vi "run_pharmaBotExp_v0.015.vi"(0 "data in":T12={"daq_ao 1"="Dev1/ao0", "daq_ai 1"="Dev1/ai0", "experiment day folder"=path "C:/multiBot/data/debug/testing", "Multiclamp init error"=0, "Multiclamp Handle Out"=10225184, "sampling rate (Hz)"=20000, "trial name"="t1"}, 1 "auto run?":bool=TRUE, 3 "which manipulator":T13(ring), 4 "HEK/slice options":enum16{"slice", "HEK"}(ring), 5 "error in":errorcluster, 6 "Validate after Experiment":bool, 7 "common cluster":T9, 11 "individual controls in":T8, 13 "images":T3={"slice image"="remote image 000000001461186C", "pipette template"="remote image 000000001461152C", "found pipette"=refnum, "pipette mask for cell tracker"=refnum, "cell images ref"=refnum}) -> (10 "Cell Looks Good?":bool=TRUE, 12 "ValidationOutputCluster":T5(array[cluster]), 14 "ValidationResults":waveform(dbl)[][](array[waveform]), 15 "ValidationPos1":T6(array[ring]), 16 "Exp. Terminated":bool, 17 "ValidationPos2":T6(array[ring]), 18 "ValidationWaveform":waveform(dbl)[](array[waveform]), 19 "error out":errorcluster)   [LabVIEW 2015] (continued)
              tunnel: w1798 -> [_ _ _ _ _ _ _ _ _ w1834 _ _ _ _ _]
              tunnel: w1797 -> [_ _ _ _ _ _ _ _ _ _ w1837 _ _ _ _]
              tunnel: w1796 -> [_ _ _ _ _ _ _ _ _ _ _ w1840 _ _ _]
              tunnel: w1795 -> [_ _ _ _ _ _ _ _ _ _ _ _ w1843 _ _]
              frame "False", Default {
              }
              frame "Single Jump" {
                n1386 = property class="TabCtl (strict)"(reference=w1811, "Value"=w1810) -> ()  [unwired: 1 in, 2 out]
                n1387 = property class="TabCtl (strict)"(reference=w1811, "Visible"=TRUE) -> ()  [unwired: 1 in, 2 out]
              }
              frame "Solution Change" {
                n1388 = property class="TabCtl (strict)"(reference=w1814, "Visible"=TRUE) -> ()  [unwired: 1 in, 2 out]
                n1389 = property class="TabCtl (strict)"(reference=w1814, "Value"=w1813) -> ()  [unwired: 1 in, 2 out]
              }
              frame "Voltage Step" {
                n1390 = property class="TabCtl (strict)"(reference=w1817, "Value"=w1816) -> ()  [unwired: 1 in, 2 out]
                n1391 = property class="TabCtl (strict)"(reference=w1817, "Visible"=TRUE) -> ()  [unwired: 1 in, 2 out]
              }
              frame "Voltage Ramp" {
                n1392 = property class="TabCtl (strict)"(reference=w1820, "Value"=w1819) -> ()  [unwired: 1 in, 2 out]
                n1393 = property class="TabCtl (strict)"(reference=w1820, "Visible"=TRUE) -> ()  [unwired: 1 in, 2 out]
              }
              frame "Voltage Pulse" {
                n1394 = property class="TabCtl (strict)"(reference=w1823, "Value"=w1822) -> ()  [unwired: 1 in, 2 out]
                n1395 = property class="TabCtl (strict)"(reference=w1823, "Visible"=TRUE) -> ()  [unwired: 1 in, 2 out]
              }
              frame "Jump Train" {
                n1396 = property class="TabCtl (strict)"(reference=w1826, "Value"=w1825) -> ()  [unwired: 1 in, 2 out]
                n1397 = property class="TabCtl (strict)"(reference=w1826, "Visible"=TRUE) -> ()  [unwired: 1 in, 2 out]
              }
              frame "Paired Pulse" {
                n1398 = property class="TabCtl (strict)"(reference=w1829, "Value"=w1828) -> ()  [unwired: 1 in, 2 out]
                n1399 = property class="TabCtl (strict)"(reference=w1829, "Visible"=TRUE) -> ()  [unwired: 1 in, 2 out]
              }
              frame "Single Manip Jump" {
                n1400 = property class="TabCtl (strict)"(reference=w1832, "Value"=w1831) -> ()  [unwired: 1 in, 2 out]
                n1401 = property class="TabCtl (strict)"(reference=w1832, "Visible"=TRUE) -> ()  [unwired: 1 in, 2 out]
              }
              frame "Gap Free" {
                n1402 = property class="TabCtl (strict)"(reference=w1835, "Value"=w1834) -> ()  [unwired: 1 in, 2 out]
                n1403 = property class="TabCtl (strict)"(reference=w1835, "Visible"=TRUE) -> ()  [unwired: 1 in, 2 out]
              }
              frame "Gap Free Iclamp" {
                n1404 = property class="TabCtl (strict)"(reference=w1838, "Value"=w1837) -> ()  [unwired: 1 in, 2 out]
                n1405 = property class="TabCtl (strict)"(reference=w1838, "Visible"=TRUE) -> ()  [unwired: 1 in, 2 out]
              }
              frame "Current Pulse" {
                n1406 = property class="TabCtl (strict)"(reference=w1841, "Value"=w1840) -> ()  [unwired: 1 in, 2 out]
                n1407 = property class="TabCtl (strict)"(reference=w1841, "Visible"=TRUE) -> ()  [unwired: 1 in, 2 out]
              }
              frame "Current Ramp" {
                n1408 = property class="TabCtl (strict)"(reference=w1844, "Value"=w1843) -> ()  [unwired: 1 in, 2 out]
                n1409 = property class="TabCtl (strict)"(reference=w1844, "Visible"=TRUE) -> ()  [unwired: 1 in, 2 out]
              }
              frame "Multi M. Jump" {
                n1410 = property class="TabCtl (strict)"(reference=w1847, "Value"=w1846) -> ()  [unwired: 1 in, 2 out]
                n1411 = property class="TabCtl (strict)"(reference=w1847, "Visible"=TRUE) -> ()  [unwired: 1 in, 2 out]
              }
              frame "none" {
                n1412 = property class="TabCtl (strict)"(reference=w1849, "Visible"=FALSE) -> ()  [unwired: 1 in, 2 out]
              }
            }
          }
          frame "PhaseC Experiment Option" {
            n1413 = control-ref of="Experiment Selection C"() -> (w1864:refnum<vi>)
            n1414 = case shown="\"Current Ramp\"" w1865 {
              tunnel: w1864 -> [_ w1867 w1870 w1873 w1876 w1879 w1882 w1885 w1888 w1891 w1894 w1897 w1900 w1903 w1905]
              tunnel: w1863 -> [_ _ _ _ _ _ _ _ _ _ _ _ _ w1902 _]
              tunnel: w1862 -> [_ w1866 _ _ _ _ _ _ _ _ _ _ _ _ _]
              tunnel: w1861 -> [_ _ w1869 _ _ _ _ _ _ _ _ _ _ _ _]
              tunnel: w1860 -> [_ _ _ w1872 _ _ _ _ _ _ _ _ _ _ _]
              tunnel: w1859 -> [_ _ _ _ w1875 _ _ _ _ _ _ _ _ _ _]
              tunnel: w1858 -> [_ _ _ _ _ w1878 _ _ _ _ _ _ _ _ _]
              tunnel: w1857 -> [_ _ _ _ _ _ w1881 _ _ _ _ _ _ _ _]
              tunnel: w1856 -> [_ _ _ _ _ _ _ w1884 _ _ _ _ _ _ _]
              tunnel: w1855 -> [_ _ _ _ _ _ _ _ w1887 _ _ _ _ _ _]
              tunnel: w1854 -> [_ _ _ _ _ _ _ _ _ w1890 _ _ _ _ _]
              tunnel: w1853 -> [_ _ _ _ _ _ _ _ _ _ w1893 _ _ _ _]
              tunnel: w1852 -> [_ _ _ _ _ _ _ _ _ _ _ w1896 _ _ _]
              tunnel: w1851 -> [_ _ _ _ _ _ _ _ _ _ _ _ w1899 _ _]
              frame "False", Default {
              }
              frame "Single Jump" {
                n1415 = property class="TabCtl (strict)"(reference=w1867, "Value"=w1866) -> ()  [unwired: 1 in, 2 out]
                n1416 = property class="TabCtl (strict)"(reference=w1867, "Visible"=TRUE) -> ()  [unwired: 1 in, 2 out]
              }
              frame "Solution Change" {
                n1417 = property class="TabCtl (strict)"(reference=w1870, "Visible"=TRUE) -> ()  [unwired: 1 in, 2 out]
                n1418 = property class="TabCtl (strict)"(reference=w1870, "Value"=w1869) -> ()  [unwired: 1 in, 2 out]
              }
              frame "Voltage Step" {
                n1419 = property class="TabCtl (strict)"(reference=w1873, "Value"=w1872) -> ()  [unwired: 1 in, 2 out]
                n1420 = property class="TabCtl (strict)"(reference=w1873, "Visible"=TRUE) -> ()  [unwired: 1 in, 2 out]
              }
              frame "Voltage Ramp" {
                n1421 = property class="TabCtl (strict)"(reference=w1876, "Value"=w1875) -> ()  [unwired: 1 in, 2 out]
                n1422 = property class="TabCtl (strict)"(reference=w1876, "Visible"=TRUE) -> ()  [unwired: 1 in, 2 out]
              }
              frame "Voltage Pulse" {
                n1423 = property class="TabCtl (strict)"(reference=w1879, "Value"=w1878) -> ()  [unwired: 1 in, 2 out]
                n1424 = property class="TabCtl (strict)"(reference=w1879, "Visible"=TRUE) -> ()  [unwired: 1 in, 2 out]
              }
              frame "Jump Train" {
                n1425 = property class="TabCtl (strict)"(reference=w1882, "Value"=w1881) -> ()  [unwired: 1 in, 2 out]
                n1426 = property class="TabCtl (strict)"(reference=w1882, "Visible"=TRUE) -> ()  [unwired: 1 in, 2 out]
              }
              frame "Paired Pulse" {
                n1427 = property class="TabCtl (strict)"(reference=w1885, "Value"=w1884) -> ()  [unwired: 1 in, 2 out]
                n1428 = property class="TabCtl (strict)"(reference=w1885, "Visible"=TRUE) -> ()  [unwired: 1 in, 2 out]
              }
              frame "Single Manip Jump" {
                n1429 = property class="TabCtl (strict)"(reference=w1888, "Value"=w1887) -> ()  [unwired: 1 in, 2 out]
                n1430 = property class="TabCtl (strict)"(reference=w1888, "Visible"=TRUE) -> ()  [unwired: 1 in, 2 out]
              }
              frame "Gap Free" {
                n1431 = property class="TabCtl (strict)"(reference=w1891, "Value"=w1890) -> ()  [unwired: 1 in, 2 out]
                n1432 = property class="TabCtl (strict)"(reference=w1891, "Visible"=TRUE) -> ()  [unwired: 1 in, 2 out]
              }
              frame "Gap Free Iclamp" {
                n1433 = property class="TabCtl (strict)"(reference=w1894, "Value"=w1893) -> ()  [unwired: 1 in, 2 out]
                n1434 = property class="TabCtl (strict)"(reference=w1894, "Visible"=TRUE) -> ()  [unwired: 1 in, 2 out]
              }
              frame "Current Pulse" {
                n1435 = property class="TabCtl (strict)"(reference=w1897, "Value"=w1896) -> ()  [unwired: 1 in, 2 out]
                n1436 = property class="TabCtl (strict)"(reference=w1897, "Visible"=TRUE) -> ()  [unwired: 1 in, 2 out]
              }
              frame "Current Ramp" {
                n1437 = property class="TabCtl (strict)"(reference=w1900, "Value"=w1899) -> ()  [unwired: 1 in, 2 out]
                n1438 = property class="TabCtl (strict)"(reference=w1900, "Visible"=TRUE) -> ()  [unwired: 1 in, 2 out]
              }
              frame "Multi M. Jump" {
                n1439 = property class="TabCtl (strict)"(reference=w1903, "Value"=w1902) -> ()  [unwired: 1 in, 2 out]
                n1440 = property class="TabCtl (strict)"(reference=w1903, "Visible"=TRUE) -> ()  [unwired: 1 in, 2 out]
              }
              frame "none" {
                n1441 = property class="TabCtl (strict)"(reference=w1905, "Visible"=FALSE) -> ()  [unwired: 1 in, 2 out]
              }
            }
          }
          frame "PhaseD Experiment Option" {
            n1442 = control-ref of="Experiment Selection D"() -> (w1920:refnum<vi>)
            n1443 = case shown="\"Current Ramp\"" w1921 {
              tunnel: w1920 -> [_ w1923 w1926 w1929 w1932 w1935 w1938 w1941 w1944 w1947 w1950 w1953 w1956 w1959 w1961]
              tunnel: w1919 -> [_ _ _ _ _ _ _ _ _ _ _ _ _ w1958 _]
              tunnel: w1918 -> [_ w1922 _ _ _ _ _ _ _ _ _ _ _ _ _]
              tunnel: w1917 -> [_ _ w1925 _ _ _ _ _ _ _ _ _ _ _ _]
              tunnel: w1916 -> [_ _ _ w1928 _ _ _ _ _ _ _ _ _ _ _]
              tunnel: w1915 -> [_ _ _ _ w1931 _ _ _ _ _ _ _ _ _ _]
              tunnel: w1914 -> [_ _ _ _ _ w1934 _ _ _ _ _ _ _ _ _]
              tunnel: w1913 -> [_ _ _ _ _ _ w1937 _ _ _ _ _ _ _ _]
              tunnel: w1912 -> [_ _ _ _ _ _ _ w1940 _ _ _ _ _ _ _]
              tunnel: w1911 -> [_ _ _ _ _ _ _ _ w1943 _ _ _ _ _ _]
              tunnel: w1910 -> [_ _ _ _ _ _ _ _ _ w1946 _ _ _ _ _]
              tunnel: w1909 -> [_ _ _ _ _ _ _ _ _ _ w1949 _ _ _ _]
              tunnel: w1908 -> [_ _ _ _ _ _ _ _ _ _ _ w1952 _ _ _]
              tunnel: w1907 -> [_ _ _ _ _ _ _ _ _ _ _ _ w1955 _ _]
              frame "False", Default {
              }
              frame "Single Jump" {
                n1444 = property class="TabCtl (strict)"(reference=w1923, "Value"=w1922) -> ()  [unwired: 1 in, 2 out]
                n1445 = property class="TabCtl (strict)"(reference=w1923, "Visible"=TRUE) -> ()  [unwired: 1 in, 2 out]
              }
              frame "Solution Change" {
                n1446 = property class="TabCtl (strict)"(reference=w1926, "Visible"=TRUE) -> ()  [unwired: 1 in, 2 out]
                n1447 = property class="TabCtl (strict)"(reference=w1926, "Value"=w1925) -> ()  [unwired: 1 in, 2 out]
              }
              frame "Voltage Step" {
                n1448 = property class="TabCtl (strict)"(reference=w1929, "Value"=w1928) -> ()  [unwired: 1 in, 2 out]
                n1449 = property class="TabCtl (strict)"(reference=w1929, "Visible"=TRUE) -> ()  [unwired: 1 in, 2 out]
              }
              frame "Voltage Ramp" {
                n1450 = property class="TabCtl (strict)"(reference=w1932, "Value"=w1931) -> ()  [unwired: 1 in, 2 out]
                n1451 = property class="TabCtl (strict)"(reference=w1932, "Visible"=TRUE) -> ()  [unwired: 1 in, 2 out]
              }
              frame "Voltage Pulse" {
                n1452 = property class="TabCtl (strict)"(reference=w1935, "Value"=w1934) -> ()  [unwired: 1 in, 2 out]
                n1453 = property class="TabCtl (strict)"(reference=w1935, "Visible"=TRUE) -> ()  [unwired: 1 in, 2 out]
              }
              frame "Jump Train" {
                n1454 = property class="TabCtl (strict)"(reference=w1938, "Value"=w1937) -> ()  [unwired: 1 in, 2 out]
                n1455 = property class="TabCtl (strict)"(reference=w1938, "Visible"=TRUE) -> ()  [unwired: 1 in, 2 out]
              }
              frame "Paired Pulse" {
                n1456 = property class="TabCtl (strict)"(reference=w1941, "Value"=w1940) -> ()  [unwired: 1 in, 2 out]
                n1457 = property class="TabCtl (strict)"(reference=w1941, "Visible"=TRUE) -> ()  [unwired: 1 in, 2 out]
              }
              frame "Single Manip Jump" {
                n1458 = property class="TabCtl (strict)"(reference=w1944, "Value"=w1943) -> ()  [unwired: 1 in, 2 out]
                n1459 = property class="TabCtl (strict)"(reference=w1944, "Visible"=TRUE) -> ()  [unwired: 1 in, 2 out]
              }
              frame "Gap Free" {
                n1460 = property class="TabCtl (strict)"(reference=w1947, "Value"=w1946) -> ()  [unwired: 1 in, 2 out]
                n1461 = property class="TabCtl (strict)"(reference=w1947, "Visible"=TRUE) -> ()  [unwired: 1 in, 2 out]
              }
              frame "Gap Free Iclamp" {
                n1462 = property class="TabCtl (strict)"(reference=w1950, "Value"=w1949) -> ()  [unwired: 1 in, 2 out]
                n1463 = property class="TabCtl (strict)"(reference=w1950, "Visible"=TRUE) -> ()  [unwired: 1 in, 2 out]
              }
              frame "Current Pulse" {
                n1464 = property class="TabCtl (strict)"(reference=w1953, "Value"=w1952) -> ()  [unwired: 1 in, 2 out]
                n1465 = property class="TabCtl (strict)"(reference=w1953, "Visible"=TRUE) -> ()  [unwired: 1 in, 2 out]
              }
              frame "Current Ramp" {
                n1466 = property class="TabCtl (strict)"(reference=w1956, "Value"=w1955) -> ()  [unwired: 1 in, 2 out]
                n1467 = property class="TabCtl (strict)"(reference=w1956, "Visible"=TRUE) -> ()  [unwired: 1 in, 2 out]
              }
              frame "Multi M. Jump" {
                n1468 = property class="TabCtl (strict)"(reference=w1959, "Value"=w1958) -> ()  [unwired: 1 in, 2 out]
                n1469 = property class="TabCtl (strict)"(reference=w1959, "Visible"=TRUE) -> ()  [unwired: 1 in, 2 out]
              }
              frame "none" {
                n1470 = property class="TabCtl (strict)"(reference=w1961, "Visible"=FALSE) -> ()  [unwired: 1 in, 2 out]
              }
            }
          }
          frame "PhaseE Experiment Option" {
            n1471 = control-ref of="Experiment Selection E"() -> (w1976:refnum<vi>)
            n1472 = case shown="\"Current Ramp\"" w1977 {
              tunnel: w1976 -> [_ w1979 w1982 w1985 w1988 w1991 w1994 w1997 w2000 w2003 w2006 w2009 w2012 w2015 w2017]
              tunnel: w1975 -> [_ _ _ _ _ _ _ _ _ _ _ _ _ w2014 _]
              tunnel: w1974 -> [_ w1978 _ _ _ _ _ _ _ _ _ _ _ _ _]
              tunnel: w1973 -> [_ _ w1981 _ _ _ _ _ _ _ _ _ _ _ _]
              tunnel: w1972 -> [_ _ _ w1984 _ _ _ _ _ _ _ _ _ _ _]
              tunnel: w1971 -> [_ _ _ _ w1987 _ _ _ _ _ _ _ _ _ _]
              tunnel: w1970 -> [_ _ _ _ _ w1990 _ _ _ _ _ _ _ _ _]
              tunnel: w1969 -> [_ _ _ _ _ _ w1993 _ _ _ _ _ _ _ _]
              tunnel: w1968 -> [_ _ _ _ _ _ _ w1996 _ _ _ _ _ _ _]
              tunnel: w1967 -> [_ _ _ _ _ _ _ _ w1999 _ _ _ _ _ _]
              tunnel: w1966 -> [_ _ _ _ _ _ _ _ _ w2002 _ _ _ _ _]
              tunnel: w1965 -> [_ _ _ _ _ _ _ _ _ _ w2005 _ _ _ _]
              tunnel: w1964 -> [_ _ _ _ _ _ _ _ _ _ _ w2008 _ _ _]
              tunnel: w1963 -> [_ _ _ _ _ _ _ _ _ _ _ _ w2011 _ _]
              frame "False", Default {
              }
              frame "Single Jump" {
                n1473 = property class="TabCtl (strict)"(reference=w1979, "Value"=w1978) -> ()  [unwired: 1 in, 2 out]
                n1474 = property class="TabCtl (strict)"(reference=w1979, "Visible"=TRUE) -> ()  [unwired: 1 in, 2 out]
              }
              frame "Solution Change" {
                n1475 = property class="TabCtl (strict)"(reference=w1982, "Visible"=TRUE) -> ()  [unwired: 1 in, 2 out]
                n1476 = property class="TabCtl (strict)"(reference=w1982, "Value"=w1981) -> ()  [unwired: 1 in, 2 out]
              }
              frame "Voltage Step" {
                n1477 = property class="TabCtl (strict)"(reference=w1985, "Value"=w1984) -> ()  [unwired: 1 in, 2 out]
                n1478 = property class="TabCtl (strict)"(reference=w1985, "Visible"=TRUE) -> ()  [unwired: 1 in, 2 out]
              }
              frame "Voltage Ramp" {
                n1479 = property class="TabCtl (strict)"(reference=w1988, "Value"=w1987) -> ()  [unwired: 1 in, 2 out]
                n1480 = property class="TabCtl (strict)"(reference=w1988, "Visible"=TRUE) -> ()  [unwired: 1 in, 2 out]
              }
              frame "Voltage Pulse" {
                n1481 = property class="TabCtl (strict)"(reference=w1991, "Value"=w1990) -> ()  [unwired: 1 in, 2 out]
                n1482 = property class="TabCtl (strict)"(reference=w1991, "Visible"=TRUE) -> ()  [unwired: 1 in, 2 out]
              }
              frame "Jump Train" {
                n1483 = property class="TabCtl (strict)"(reference=w1994, "Value"=w1993) -> ()  [unwired: 1 in, 2 out]
                n1484 = property class="TabCtl (strict)"(reference=w1994, "Visible"=TRUE) -> ()  [unwired: 1 in, 2 out]
              }
              frame "Paired Pulse" {
                n1485 = property class="TabCtl (strict)"(reference=w1997, "Value"=w1996) -> ()  [unwired: 1 in, 2 out]
                n1486 = property class="TabCtl (strict)"(reference=w1997, "Visible"=TRUE) -> ()  [unwired: 1 in, 2 out]
              }
              frame "Single Manip Jump" {
                n1487 = property class="TabCtl (strict)"(reference=w2000, "Value"=w1999) -> ()  [unwired: 1 in, 2 out]
                n1488 = property class="TabCtl (strict)"(reference=w2000, "Visible"=TRUE) -> ()  [unwired: 1 in, 2 out]
              }
              frame "Gap Free" {
                n1489 = property class="TabCtl (strict)"(reference=w2003, "Value"=w2002) -> ()  [unwired: 1 in, 2 out]
                n1490 = property class="TabCtl (strict)"(reference=w2003, "Visible"=TRUE) -> ()  [unwired: 1 in, 2 out]
              }
              frame "Gap Free Iclamp" {
                n1491 = property class="TabCtl (strict)"(reference=w2006, "Value"=w2005) -> ()  [unwired: 1 in, 2 out]
                n1492 = property class="TabCtl (strict)"(reference=w2006, "Visible"=TRUE) -> ()  [unwired: 1 in, 2 out]
              }
              frame "Current Pulse" {
                n1493 = property class="TabCtl (strict)"(reference=w2009, "Value"=w2008) -> ()  [unwired: 1 in, 2 out]
                n1494 = property class="TabCtl (strict)"(reference=w2009, "Visible"=TRUE) -> ()  [unwired: 1 in, 2 out]
              }
              frame "Current Ramp" {
                n1495 = property class="TabCtl (strict)"(reference=w2012, "Value"=w2011) -> ()  [unwired: 1 in, 2 out]
                n1496 = property class="TabCtl (strict)"(reference=w2012, "Visible"=TRUE) -> ()  [unwired: 1 in, 2 out]
              }
              frame "Multi M. Jump" {
                n1497 = property class="TabCtl (strict)"(reference=w2015, "Value"=w2014) -> ()  [unwired: 1 in, 2 out]
                n1498 = property class="TabCtl (strict)"(reference=w2015, "Visible"=TRUE) -> ()  [unwired: 1 in, 2 out]
              }
              frame "none" {
                n1499 = property class="TabCtl (strict)"(reference=w2017, "Visible"=FALSE) -> ()  [unwired: 1 in, 2 out]
              }
            }
          }
          frame "PhaseF Experiment Option" {
            n1500 = control-ref of="Experiment Selection F"() -> (w2032:refnum<vi>)
            n1501 = case shown="\"Current Ramp\"" w2033 {
              tunnel: w2032 -> [_ w2035 w2038 w2041 w2044 w2047 w2050 w2053 w2056 w2059 w2062 w2065 w2068 w2071 w2073]
              tunnel: w2031 -> [_ _ _ _ _ _ _ _ _ _ _ _ _ w2070 _]
              tunnel: w2030 -> [_ w2034 _ _ _ _ _ _ _ _ _ _ _ _ _]
              tunnel: w2029 -> [_ _ w2037 _ _ _ _ _ _ _ _ _ _ _ _]
              tunnel: w2028 -> [_ _ _ w2040 _ _ _ _ _ _ _ _ _ _ _]
              tunnel: w2027 -> [_ _ _ _ w2043 _ _ _ _ _ _ _ _ _ _]
              tunnel: w2026 -> [_ _ _ _ _ w2046 _ _ _ _ _ _ _ _ _]
              tunnel: w2025 -> [_ _ _ _ _ _ w2049 _ _ _ _ _ _ _ _]
              tunnel: w2024 -> [_ _ _ _ _ _ _ w2052 _ _ _ _ _ _ _]
              tunnel: w2023 -> [_ _ _ _ _ _ _ _ w2055 _ _ _ _ _ _]
              tunnel: w2022 -> [_ _ _ _ _ _ _ _ _ w2058 _ _ _ _ _]
              tunnel: w2021 -> [_ _ _ _ _ _ _ _ _ _ w2061 _ _ _ _]
              tunnel: w2020 -> [_ _ _ _ _ _ _ _ _ _ _ w2064 _ _ _]
              tunnel: w2019 -> [_ _ _ _ _ _ _ _ _ _ _ _ w2067 _ _]
              frame "False", Default {
              }
              frame "Single Jump" {
                n1502 = property class="TabCtl (strict)"(reference=w2035, "Value"=w2034) -> ()  [unwired: 1 in, 2 out]
                n1503 = property class="TabCtl (strict)"(reference=w2035, "Visible"=TRUE) -> ()  [unwired: 1 in, 2 out]
              }
              frame "Solution Change" {
                n1504 = property class="TabCtl (strict)"(reference=w2038, "Visible"=TRUE) -> ()  [unwired: 1 in, 2 out]
                n1505 = property class="TabCtl (strict)"(reference=w2038, "Value"=w2037) -> ()  [unwired: 1 in, 2 out]
              }
              frame "Voltage Step" {
                n1506 = property class="TabCtl (strict)"(reference=w2041, "Value"=w2040) -> ()  [unwired: 1 in, 2 out]
                n1507 = property class="TabCtl (strict)"(reference=w2041, "Visible"=TRUE) -> ()  [unwired: 1 in, 2 out]
              }
              frame "Voltage Ramp" {
                n1508 = property class="TabCtl (strict)"(reference=w2044, "Value"=w2043) -> ()  [unwired: 1 in, 2 out]
                n1509 = property class="TabCtl (strict)"(reference=w2044, "Visible"=TRUE) -> ()  [unwired: 1 in, 2 out]
              }
              frame "Voltage Pulse" {
                n1510 = property class="TabCtl (strict)"(reference=w2047, "Value"=w2046) -> ()  [unwired: 1 in, 2 out]
                n1511 = property class="TabCtl (strict)"(reference=w2047, "Visible"=TRUE) -> ()  [unwired: 1 in, 2 out]
              }
              frame "Jump Train" {
                n1512 = property class="TabCtl (strict)"(reference=w2050, "Value"=w2049) -> ()  [unwired: 1 in, 2 out]
                n1513 = property class="TabCtl (strict)"(reference=w2050, "Visible"=TRUE) -> ()  [unwired: 1 in, 2 out]
              }
              frame "Paired Pulse" {
                n1514 = property class="TabCtl (strict)"(reference=w2053, "Value"=w2052) -> ()  [unwired: 1 in, 2 out]
                n1515 = property class="TabCtl (strict)"(reference=w2053, "Visible"=TRUE) -> ()  [unwired: 1 in, 2 out]
              }
              frame "Single Manip Jump" {
                n1516 = property class="TabCtl (strict)"(reference=w2056, "Value"=w2055) -> ()  [unwired: 1 in, 2 out]
                n1517 = property class="TabCtl (strict)"(reference=w2056, "Visible"=TRUE) -> ()  [unwired: 1 in, 2 out]
              }
              frame "Gap Free" {
                n1518 = property class="TabCtl (strict)"(reference=w2059, "Value"=w2058) -> ()  [unwired: 1 in, 2 out]
                n1519 = property class="TabCtl (strict)"(reference=w2059, "Visible"=TRUE) -> ()  [unwired: 1 in, 2 out]
              }
              frame "Gap Free Iclamp" {
                n1520 = property class="TabCtl (strict)"(reference=w2062, "Value"=w2061) -> ()  [unwired: 1 in, 2 out]
                n1521 = property class="TabCtl (strict)"(reference=w2062, "Visible"=TRUE) -> ()  [unwired: 1 in, 2 out]
              }
              frame "Current Pulse" {
                n1522 = property class="TabCtl (strict)"(reference=w2065, "Value"=w2064) -> ()  [unwired: 1 in, 2 out]
                n1523 = property class="TabCtl (strict)"(reference=w2065, "Visible"=TRUE) -> ()  [unwired: 1 in, 2 out]
              }
              frame "Current Ramp" {
                n1524 = property class="TabCtl (strict)"(reference=w2068, "Value"=w2067) -> ()  [unwired: 1 in, 2 out]
                n1525 = property class="TabCtl (strict)"(reference=w2068, "Visible"=TRUE) -> ()  [unwired: 1 in, 2 out]
              }
              frame "Multi M. Jump" {
                n1526 = property class="TabCtl (strict)"(reference=w2071, "Value"=w2070) -> ()  [unwired: 1 in, 2 out]
                n1527 = property class="TabCtl (strict)"(reference=w2071, "Visible"=TRUE) -> ()  [unwired: 1 in, 2 out]
              }
              frame "none" {
                n1528 = property class="TabCtl (strict)"(reference=w2073, "Visible"=FALSE) -> ()  [unwired: 1 in, 2 out]
              }
            }
          }
          frame "PhaseG Experiment Option" {
            n1529 = control-ref of="Experiment Selection G"() -> (w2088:refnum<vi>)
            n1530 = case shown="\"Current Ramp\"" w2089 {
              tunnel: w2088 -> [_ w2091 w2094 w2097 w2100 w2103 w2106 w2109 w2112 w2115 w2118 w2121 w2124 w2127 w2129]
              tunnel: w2087 -> [_ _ _ _ _ _ _ _ _ _ _ _ _ w2126 _]
              tunnel: w2086 -> [_ w2090 _ _ _ _ _ _ _ _ _ _ _ _ _]
              tunnel: w2085 -> [_ _ w2093 _ _ _ _ _ _ _ _ _ _ _ _]
              tunnel: w2084 -> [_ _ _ w2096 _ _ _ _ _ _ _ _ _ _ _]
              tunnel: w2083 -> [_ _ _ _ w2099 _ _ _ _ _ _ _ _ _ _]
              tunnel: w2082 -> [_ _ _ _ _ w2102 _ _ _ _ _ _ _ _ _]
              tunnel: w2081 -> [_ _ _ _ _ _ w2105 _ _ _ _ _ _ _ _]
              tunnel: w2080 -> [_ _ _ _ _ _ _ w2108 _ _ _ _ _ _ _]
              tunnel: w2079 -> [_ _ _ _ _ _ _ _ w2111 _ _ _ _ _ _]
              tunnel: w2078 -> [_ _ _ _ _ _ _ _ _ w2114 _ _ _ _ _]
              tunnel: w2077 -> [_ _ _ _ _ _ _ _ _ _ w2117 _ _ _ _]
              tunnel: w2076 -> [_ _ _ _ _ _ _ _ _ _ _ w2120 _ _ _]
              tunnel: w2075 -> [_ _ _ _ _ _ _ _ _ _ _ _ w2123 _ _]
              frame "False", Default {
              }
              frame "Single Jump" {
                n1531 = property class="TabCtl (strict)"(reference=w2091, "Value"=w2090) -> ()  [unwired: 1 in, 2 out]
                n1532 = property class="TabCtl (strict)"(reference=w2091, "Visible"=TRUE) -> ()  [unwired: 1 in, 2 out]
              }
              frame "Solution Change" {
                n1533 = property class="TabCtl (strict)"(reference=w2094, "Visible"=TRUE) -> ()  [unwired: 1 in, 2 out]
                n1534 = property class="TabCtl (strict)"(reference=w2094, "Value"=w2093) -> ()  [unwired: 1 in, 2 out]
              }
              frame "Voltage Step" {
                n1535 = property class="TabCtl (strict)"(reference=w2097, "Value"=w2096) -> ()  [unwired: 1 in, 2 out]
                n1536 = property class="TabCtl (strict)"(reference=w2097, "Visible"=TRUE) -> ()  [unwired: 1 in, 2 out]
              }
              frame "Voltage Ramp" {
                n1537 = property class="TabCtl (strict)"(reference=w2100, "Value"=w2099) -> ()  [unwired: 1 in, 2 out]
                n1538 = property class="TabCtl (strict)"(reference=w2100, "Visible"=TRUE) -> ()  [unwired: 1 in, 2 out]
              }
              frame "Voltage Pulse" {
                n1539 = property class="TabCtl (strict)"(reference=w2103, "Value"=w2102) -> ()  [unwired: 1 in, 2 out]
                n1540 = property class="TabCtl (strict)"(reference=w2103, "Visible"=TRUE) -> ()  [unwired: 1 in, 2 out]
              }
              frame "Jump Train" {
                n1541 = property class="TabCtl (strict)"(reference=w2106, "Value"=w2105) -> ()  [unwired: 1 in, 2 out]
                n1542 = property class="TabCtl (strict)"(reference=w2106, "Visible"=TRUE) -> ()  [unwired: 1 in, 2 out]
              }
              frame "Paired Pulse" {
                n1543 = property class="TabCtl (strict)"(reference=w2109, "Value"=w2108) -> ()  [unwired: 1 in, 2 out]
                n1544 = property class="TabCtl (strict)"(reference=w2109, "Visible"=TRUE) -> ()  [unwired: 1 in, 2 out]
              }
              frame "Single Manip Jump" {
                n1545 = property class="TabCtl (strict)"(reference=w2112, "Value"=w2111) -> ()  [unwired: 1 in, 2 out]
                n1546 = property class="TabCtl (strict)"(reference=w2112, "Visible"=TRUE) -> ()  [unwired: 1 in, 2 out]
              }
              frame "Gap Free" {
                n1547 = property class="TabCtl (strict)"(reference=w2115, "Value"=w2114) -> ()  [unwired: 1 in, 2 out]
                n1548 = property class="TabCtl (strict)"(reference=w2115, "Visible"=TRUE) -> ()  [unwired: 1 in, 2 out]
              }
              frame "Gap Free Iclamp" {
                n1549 = property class="TabCtl (strict)"(reference=w2118, "Value"=w2117) -> ()  [unwired: 1 in, 2 out]
                n1550 = property class="TabCtl (strict)"(reference=w2118, "Visible"=TRUE) -> ()  [unwired: 1 in, 2 out]
              }
              frame "Current Pulse" {
                n1551 = property class="TabCtl (strict)"(reference=w2121, "Value"=w2120) -> ()  [unwired: 1 in, 2 out]
                n1552 = property class="TabCtl (strict)"(reference=w2121, "Visible"=TRUE) -> ()  [unwired: 1 in, 2 out]
              }
              frame "Current Ramp" {
                n1553 = property class="TabCtl (strict)"(reference=w2124, "Value"=w2123) -> ()  [unwired: 1 in, 2 out]
                n1554 = property class="TabCtl (strict)"(reference=w2124, "Visible"=TRUE) -> ()  [unwired: 1 in, 2 out]
              }
              frame "Multi M. Jump" {
                n1555 = property class="TabCtl (strict)"(reference=w2127, "Value"=w2126) -> ()  [unwired: 1 in, 2 out]
                n1556 = property class="TabCtl (strict)"(reference=w2127, "Visible"=TRUE) -> ()  [unwired: 1 in, 2 out]
              }
              frame "none" {
                n1557 = property class="TabCtl (strict)"(reference=w2129, "Visible"=FALSE) -> ()  [unwired: 1 in, 2 out]
              }
            }
          }
          frame "PhaseH Experiment Option" {
            n1558 = control-ref of="Experiment Selection H"() -> (w2144:refnum<vi>)
            n1559 = case shown="\"Current Ramp\"" w2145 {
              tunnel: w2144 -> [_ w2147 w2150 w2153 w2156 w2159 w2162 w2165 w2168 w2171 w2174 w2177 w2180 w2183 w2185]
              tunnel: w2143 -> [_ _ _ _ _ _ _ _ _ _ _ _ _ w2182 _]
              tunnel: w2142 -> [_ w2146 _ _ _ _ _ _ _ _ _ _ _ _ _]
              tunnel: w2141 -> [_ _ w2149 _ _ _ _ _ _ _ _ _ _ _ _]
              tunnel: w2140 -> [_ _ _ w2152 _ _ _ _ _ _ _ _ _ _ _]
              tunnel: w2139 -> [_ _ _ _ w2155 _ _ _ _ _ _ _ _ _ _]
              tunnel: w2138 -> [_ _ _ _ _ w2158 _ _ _ _ _ _ _ _ _]
              tunnel: w2137 -> [_ _ _ _ _ _ w2161 _ _ _ _ _ _ _ _]
              tunnel: w2136 -> [_ _ _ _ _ _ _ w2164 _ _ _ _ _ _ _]
              tunnel: w2135 -> [_ _ _ _ _ _ _ _ w2167 _ _ _ _ _ _]
              tunnel: w2134 -> [_ _ _ _ _ _ _ _ _ w2170 _ _ _ _ _]
              tunnel: w2133 -> [_ _ _ _ _ _ _ _ _ _ w2173 _ _ _ _]
              tunnel: w2132 -> [_ _ _ _ _ _ _ _ _ _ _ w2176 _ _ _]
              tunnel: w2131 -> [_ _ _ _ _ _ _ _ _ _ _ _ w2179 _ _]
              frame "False", Default {
              }
              frame "Single Jump" {
                n1560 = property class="TabCtl (strict)"(reference=w2147, "Value"=w2146) -> ()  [unwired: 1 in, 2 out]
                n1561 = property class="TabCtl (strict)"(reference=w2147, "Visible"=TRUE) -> ()  [unwired: 1 in, 2 out]
              }
              frame "Solution Change" {
                n1562 = property class="TabCtl (strict)"(reference=w2150, "Visible"=TRUE) -> ()  [unwired: 1 in, 2 out]
                n1563 = property class="TabCtl (strict)"(reference=w2150, "Value"=w2149) -> ()  [unwired: 1 in, 2 out]
              }
              frame "Voltage Step" {
                n1564 = property class="TabCtl (strict)"(reference=w2153, "Value"=w2152) -> ()  [unwired: 1 in, 2 out]
                n1565 = property class="TabCtl (strict)"(reference=w2153, "Visible"=TRUE) -> ()  [unwired: 1 in, 2 out]
              }
              frame "Voltage Ramp" {
                n1566 = property class="TabCtl (strict)"(reference=w2156, "Value"=w2155) -> ()  [unwired: 1 in, 2 out]
                n1567 = property class="TabCtl (strict)"(reference=w2156, "Visible"=TRUE) -> ()  [unwired: 1 in, 2 out]
              }
              frame "Voltage Pulse" {
                n1568 = property class="TabCtl (strict)"(reference=w2159, "Value"=w2158) -> ()  [unwired: 1 in, 2 out]
                n1569 = property class="TabCtl (strict)"(reference=w2159, "Visible"=TRUE) -> ()  [unwired: 1 in, 2 out]
              }
              frame "Jump Train" {
                n1570 = property class="TabCtl (strict)"(reference=w2162, "Value"=w2161) -> ()  [unwired: 1 in, 2 out]
                n1571 = property class="TabCtl (strict)"(reference=w2162, "Visible"=TRUE) -> ()  [unwired: 1 in, 2 out]
              }
              frame "Paired Pulse" {
                n1572 = property class="TabCtl (strict)"(reference=w2165, "Value"=w2164) -> ()  [unwired: 1 in, 2 out]
                n1573 = property class="TabCtl (strict)"(reference=w2165, "Visible"=TRUE) -> ()  [unwired: 1 in, 2 out]
              }
              frame "Single Manip Jump" {
                n1574 = property class="TabCtl (strict)"(reference=w2168, "Value"=w2167) -> ()  [unwired: 1 in, 2 out]
                n1575 = property class="TabCtl (strict)"(reference=w2168, "Visible"=TRUE) -> ()  [unwired: 1 in, 2 out]
              }
              frame "Gap Free" {
                n1576 = property class="TabCtl (strict)"(reference=w2171, "Value"=w2170) -> ()  [unwired: 1 in, 2 out]
                n1577 = property class="TabCtl (strict)"(reference=w2171, "Visible"=TRUE) -> ()  [unwired: 1 in, 2 out]
              }
              frame "Gap Free Iclamp" {
                n1578 = property class="TabCtl (strict)"(reference=w2174, "Value"=w2173) -> ()  [unwired: 1 in, 2 out]
                n1579 = property class="TabCtl (strict)"(reference=w2174, "Visible"=TRUE) -> ()  [unwired: 1 in, 2 out]
              }
              frame "Current Pulse" {
                n1580 = property class="TabCtl (strict)"(reference=w2177, "Value"=w2176) -> ()  [unwired: 1 in, 2 out]
                n1581 = property class="TabCtl (strict)"(reference=w2177, "Visible"=TRUE) -> ()  [unwired: 1 in, 2 out]
              }
              frame "Current Ramp" {
                n1582 = property class="TabCtl (strict)"(reference=w2180, "Value"=w2179) -> ()  [unwired: 1 in, 2 out]
                n1583 = property class="TabCtl (strict)"(reference=w2180, "Visible"=TRUE) -> ()  [unwired: 1 in, 2 out]
              }
              frame "Multi M. Jump" {
                n1584 = property class="TabCtl (strict)"(reference=w2183, "Value"=w2182) -> ()  [unwired: 1 in, 2 out]
                n1585 = property class="TabCtl (strict)"(reference=w2183, "Visible"=TRUE) -> ()  [unwired: 1 in, 2 out]
              }
              frame "none" {
                n1586 = property class="TabCtl (strict)"(reference=w2185, "Visible"=FALSE) -> ()  [unwired: 1 in, 2 out]
              }
            }
          }
          frame "PhaseI Experiment Option" {
            n1587 = control-ref of="Experiment Selection I"() -> (w2200:refnum<vi>)
            n1588 = case shown="\"Current Ramp\"" w2201 {
              tunnel: w2200 -> [_ w2203 w2206 w2209 w2212 w2215 w2218 w2221 w2224 w2227 w2230 w2233 w2236 w2239 w2241]
              tunnel: w2199 -> [_ _ _ _ _ _ _ _ _ _ _ _ _ w2238 _]
              tunnel: w2198 -> [_ w2202 _ _ _ _ _ _ _ _ _ _ _ _ _]
              tunnel: w2197 -> [_ _ w2205 _ _ _ _ _ _ _ _ _ _ _ _]
              tunnel: w2196 -> [_ _ _ w2208 _ _ _ _ _ _ _ _ _ _ _]
              tunnel: w2195 -> [_ _ _ _ w2211 _ _ _ _ _ _ _ _ _ _]
              tunnel: w2194 -> [_ _ _ _ _ w2214 _ _ _ _ _ _ _ _ _]
              tunnel: w2193 -> [_ _ _ _ _ _ w2217 _ _ _ _ _ _ _ _]
              tunnel: w2192 -> [_ _ _ _ _ _ _ w2220 _ _ _ _ _ _ _]
              tunnel: w2191 -> [_ _ _ _ _ _ _ _ w2223 _ _ _ _ _ _]
              tunnel: w2190 -> [_ _ _ _ _ _ _ _ _ w2226 _ _ _ _ _]
              tunnel: w2189 -> [_ _ _ _ _ _ _ _ _ _ w2229 _ _ _ _]
              tunnel: w2188 -> [_ _ _ _ _ _ _ _ _ _ _ w2232 _ _ _]
              tunnel: w2187 -> [_ _ _ _ _ _ _ _ _ _ _ _ w2235 _ _]
              frame "False", Default {
              }
              frame "Single Jump" {
                n1589 = property class="TabCtl (strict)"(reference=w2203, "Value"=w2202) -> ()  [unwired: 1 in, 2 out]
                n1590 = property class="TabCtl (strict)"(reference=w2203, "Visible"=TRUE) -> ()  [unwired: 1 in, 2 out]
              }
              frame "Solution Change" {
                n1591 = property class="TabCtl (strict)"(reference=w2206, "Visible"=TRUE) -> ()  [unwired: 1 in, 2 out]
                n1592 = property class="TabCtl (strict)"(reference=w2206, "Value"=w2205) -> ()  [unwired: 1 in, 2 out]
              }
              frame "Voltage Step" {
                n1593 = property class="TabCtl (strict)"(reference=w2209, "Value"=w2208) -> ()  [unwired: 1 in, 2 out]
                n1594 = property class="TabCtl (strict)"(reference=w2209, "Visible"=TRUE) -> ()  [unwired: 1 in, 2 out]
              }
              frame "Voltage Ramp" {
                n1595 = property class="TabCtl (strict)"(reference=w2212, "Value"=w2211) -> ()  [unwired: 1 in, 2 out]
                n1596 = property class="TabCtl (strict)"(reference=w2212, "Visible"=TRUE) -> ()  [unwired: 1 in, 2 out]
              }
              frame "Voltage Pulse" {
                n1597 = property class="TabCtl (strict)"(reference=w2215, "Value"=w2214) -> ()  [unwired: 1 in, 2 out]
                n1598 = property class="TabCtl (strict)"(reference=w2215, "Visible"=TRUE) -> ()  [unwired: 1 in, 2 out]
              }
              frame "Jump Train" {
                n1599 = property class="TabCtl (strict)"(reference=w2218, "Value"=w2217) -> ()  [unwired: 1 in, 2 out]
                n1600 = property class="TabCtl (strict)"(reference=w2218, "Visible"=TRUE) -> ()  [unwired: 1 in, 2 out]
              }
              frame "Paired Pulse" {
                n1601 = property class="TabCtl (strict)"(reference=w2221, "Value"=w2220) -> ()  [unwired: 1 in, 2 out]
                n1602 = property class="TabCtl (strict)"(reference=w2221, "Visible"=TRUE) -> ()  [unwired: 1 in, 2 out]
              }
              frame "Single Manip Jump" {
                n1603 = property class="TabCtl (strict)"(reference=w2224, "Value"=w2223) -> ()  [unwired: 1 in, 2 out]
                n1604 = property class="TabCtl (strict)"(reference=w2224, "Visible"=TRUE) -> ()  [unwired: 1 in, 2 out]
              }
              frame "Gap Free" {
                n1605 = property class="TabCtl (strict)"(reference=w2227, "Value"=w2226) -> ()  [unwired: 1 in, 2 out]
                n1606 = property class="TabCtl (strict)"(reference=w2227, "Visible"=TRUE) -> ()  [unwired: 1 in, 2 out]
              }
              frame "Gap Free Iclamp" {
                n1607 = property class="TabCtl (strict)"(reference=w2230, "Value"=w2229) -> ()  [unwired: 1 in, 2 out]
                n1608 = property class="TabCtl (strict)"(reference=w2230, "Visible"=TRUE) -> ()  [unwired: 1 in, 2 out]
              }
              frame "Current Pulse" {
                n1609 = property class="TabCtl (strict)"(reference=w2233, "Value"=w2232) -> ()  [unwired: 1 in, 2 out]
                n1610 = property class="TabCtl (strict)"(reference=w2233, "Visible"=TRUE) -> ()  [unwired: 1 in, 2 out]
              }
              frame "Current Ramp" {
                n1611 = property class="TabCtl (strict)"(reference=w2236, "Value"=w2235) -> ()  [unwired: 1 in, 2 out]
                n1612 = property class="TabCtl (strict)"(reference=w2236, "Visible"=TRUE) -> ()  [unwired: 1 in, 2 out]
              }
              frame "Multi M. Jump" {
                n1613 = property class="TabCtl (strict)"(reference=w2239, "Value"=w2238) -> ()  [unwired: 1 in, 2 out]
                n1614 = property class="TabCtl (strict)"(reference=w2239, "Visible"=TRUE) -> ()  [unwired: 1 in, 2 out]
              }
              frame "none" {
                n1615 = property class="TabCtl (strict)"(reference=w2241, "Visible"=FALSE) -> ()  [unwired: 1 in, 2 out]
              }
            }
          }
          frame "PhaseJ Experiment Option" {
            n1616 = control-ref of="Experiment Selection J"() -> (w2256:refnum<vi>)
            n1617 = case shown="\"Current Ramp\"" w2257 {
              tunnel: w2256 -> [_ w2259 w2262 w2265 w2268 w2271 w2274 w2277 w2280 w2283 w2286 w2289 w2292 w2295 w2297]
              tunnel: w2255 -> [_ _ _ _ _ _ _ _ _ _ _ _ _ w2294 _]
              tunnel: w2254 -> [_ w2258 _ _ _ _ _ _ _ _ _ _ _ _ _]
              tunnel: w2253 -> [_ _ w2261 _ _ _ _ _ _ _ _ _ _ _ _]
              tunnel: w2252 -> [_ _ _ w2264 _ _ _ _ _ _ _ _ _ _ _]
              tunnel: w2251 -> [_ _ _ _ w2267 _ _ _ _ _ _ _ _ _ _]
              tunnel: w2250 -> [_ _ _ _ _ w2270 _ _ _ _ _ _ _ _ _]
              tunnel: w2249 -> [_ _ _ _ _ _ w2273 _ _ _ _ _ _ _ _]
              tunnel: w2248 -> [_ _ _ _ _ _ _ w2276 _ _ _ _ _ _ _]
              tunnel: w2247 -> [_ _ _ _ _ _ _ _ w2279 _ _ _ _ _ _]
              tunnel: w2246 -> [_ _ _ _ _ _ _ _ _ w2282 _ _ _ _ _]
              tunnel: w2245 -> [_ _ _ _ _ _ _ _ _ _ w2285 _ _ _ _]
              tunnel: w2244 -> [_ _ _ _ _ _ _ _ _ _ _ w2288 _ _ _]
              tunnel: w2243 -> [_ _ _ _ _ _ _ _ _ _ _ _ w2291 _ _]
              frame "False", Default {
              }
              frame "Single Jump" {
                n1618 = property class="TabCtl (strict)"(reference=w2259, "Value"=w2258) -> ()  [unwired: 1 in, 2 out]
                n1619 = property class="TabCtl (strict)"(reference=w2259, "Visible"=TRUE) -> ()  [unwired: 1 in, 2 out]
              }
              frame "Solution Change" {
                n1620 = property class="TabCtl (strict)"(reference=w2262, "Visible"=TRUE) -> ()  [unwired: 1 in, 2 out]
                n1621 = property class="TabCtl (strict)"(reference=w2262, "Value"=w2261) -> ()  [unwired: 1 in, 2 out]
              }
              frame "Voltage Step" {
                n1622 = property class="TabCtl (strict)"(reference=w2265, "Value"=w2264) -> ()  [unwired: 1 in, 2 out]
                n1623 = property class="TabCtl (strict)"(reference=w2265, "Visible"=TRUE) -> ()  [unwired: 1 in, 2 out]
              }
              frame "Voltage Ramp" {
                n1624 = property class="TabCtl (strict)"(reference=w2268, "Value"=w2267) -> ()  [unwired: 1 in, 2 out]
                n1625 = property class="TabCtl (strict)"(reference=w2268, "Visible"=TRUE) -> ()  [unwired: 1 in, 2 out]
              }
              frame "Voltage Pulse" {
                n1626 = property class="TabCtl (strict)"(reference=w2271, "Value"=w2270) -> ()  [unwired: 1 in, 2 out]
                n1627 = property class="TabCtl (strict)"(reference=w2271, "Visible"=TRUE) -> ()  [unwired: 1 in, 2 out]
              }
              frame "Jump Train" {
                n1628 = property class="TabCtl (strict)"(reference=w2274, "Value"=w2273) -> ()  [unwired: 1 in, 2 out]
                n1629 = property class="TabCtl (strict)"(reference=w2274, "Visible"=TRUE) -> ()  [unwired: 1 in, 2 out]
              }
              frame "Paired Pulse" {
                n1630 = property class="TabCtl (strict)"(reference=w2277, "Value"=w2276) -> ()  [unwired: 1 in, 2 out]
                n1631 = property class="TabCtl (strict)"(reference=w2277, "Visible"=TRUE) -> ()  [unwired: 1 in, 2 out]
              }
              frame "Single Manip Jump" {
                n1632 = property class="TabCtl (strict)"(reference=w2280, "Value"=w2279) -> ()  [unwired: 1 in, 2 out]
                n1633 = property class="TabCtl (strict)"(reference=w2280, "Visible"=TRUE) -> ()  [unwired: 1 in, 2 out]
              }
              frame "Gap Free" {
                n1634 = property class="TabCtl (strict)"(reference=w2283, "Value"=w2282) -> ()  [unwired: 1 in, 2 out]
                n1635 = property class="TabCtl (strict)"(reference=w2283, "Visible"=TRUE) -> ()  [unwired: 1 in, 2 out]
              }
              frame "Gap Free Iclamp" {
                n1636 = property class="TabCtl (strict)"(reference=w2286, "Value"=w2285) -> ()  [unwired: 1 in, 2 out]
                n1637 = property class="TabCtl (strict)"(reference=w2286, "Visible"=TRUE) -> ()  [unwired: 1 in, 2 out]
              }
              frame "Current Pulse" {
                n1638 = property class="TabCtl (strict)"(reference=w2289, "Value"=w2288) -> ()  [unwired: 1 in, 2 out]
                n1639 = property class="TabCtl (strict)"(reference=w2289, "Visible"=TRUE) -> ()  [unwired: 1 in, 2 out]
              }
              frame "Current Ramp" {
                n1640 = property class="TabCtl (strict)"(reference=w2292, "Value"=w2291) -> ()  [unwired: 1 in, 2 out]
                n1641 = property class="TabCtl (strict)"(reference=w2292, "Visible"=TRUE) -> ()  [unwired: 1 in, 2 out]
              }
              frame "Multi M. Jump" {
                n1642 = property class="TabCtl (strict)"(reference=w2295, "Value"=w2294) -> ()  [unwired: 1 in, 2 out]
                n1643 = property class="TabCtl (strict)"(reference=w2295, "Visible"=TRUE) -> ()  [unwired: 1 in, 2 out]
              }
              frame "none" {
                n1644 = property class="TabCtl (strict)"(reference=w2297, "Visible"=FALSE) -> ()  [unwired: 1 in, 2 out]
              }
            }
          }
          frame "PhaseK Experiment Option" {
            n1645 = control-ref of="Experiment Selection K"() -> (w2312:refnum<vi>)
            n1646 = case shown="\"Current Ramp\"" w2313 {
              tunnel: w2312 -> [_ w2315 w2318 w2321 w2324 w2327 w2330 w2333 w2336 w2339 w2342 w2345 w2348 w2351 w2353]
              tunnel: w2311 -> [_ _ _ _ _ _ _ _ _ _ _ _ _ w2350 _]
              tunnel: w2310 -> [_ w2314 _ _ _ _ _ _ _ _ _ _ _ _ _]
              tunnel: w2309 -> [_ _ w2317 _ _ _ _ _ _ _ _ _ _ _ _]
              tunnel: w2308 -> [_ _ _ w2320 _ _ _ _ _ _ _ _ _ _ _]
              tunnel: w2307 -> [_ _ _ _ w2323 _ _ _ _ _ _ _ _ _ _]
              tunnel: w2306 -> [_ _ _ _ _ w2326 _ _ _ _ _ _ _ _ _]
              tunnel: w2305 -> [_ _ _ _ _ _ w2329 _ _ _ _ _ _ _ _]
              tunnel: w2304 -> [_ _ _ _ _ _ _ w2332 _ _ _ _ _ _ _]
              tunnel: w2303 -> [_ _ _ _ _ _ _ _ w2335 _ _ _ _ _ _]
              tunnel: w2302 -> [_ _ _ _ _ _ _ _ _ w2338 _ _ _ _ _]
              tunnel: w2301 -> [_ _ _ _ _ _ _ _ _ _ w2341 _ _ _ _]
              tunnel: w2300 -> [_ _ _ _ _ _ _ _ _ _ _ w2344 _ _ _]
              tunnel: w2299 -> [_ _ _ _ _ _ _ _ _ _ _ _ w2347 _ _]
              frame "False", Default {
              }
              frame "Single Jump" {
                n1647 = property class="TabCtl (strict)"(reference=w2315, "Value"=w2314) -> ()  [unwired: 1 in, 2 out]
                n1648 = property class="TabCtl (strict)"(reference=w2315, "Visible"=TRUE) -> ()  [unwired: 1 in, 2 out]
              }
              frame "Solution Change" {
                n1649 = property class="TabCtl (strict)"(reference=w2318, "Visible"=TRUE) -> ()  [unwired: 1 in, 2 out]
                n1650 = property class="TabCtl (strict)"(reference=w2318, "Value"=w2317) -> ()  [unwired: 1 in, 2 out]
              }
              frame "Voltage Step" {
                n1651 = property class="TabCtl (strict)"(reference=w2321, "Value"=w2320) -> ()  [unwired: 1 in, 2 out]
                n1652 = property class="TabCtl (strict)"(reference=w2321, "Visible"=TRUE) -> ()  [unwired: 1 in, 2 out]
              }
              frame "Voltage Ramp" {
                n1653 = property class="TabCtl (strict)"(reference=w2324, "Value"=w2323) -> ()  [unwired: 1 in, 2 out]
                n1654 = property class="TabCtl (strict)"(reference=w2324, "Visible"=TRUE) -> ()  [unwired: 1 in, 2 out]
              }
              frame "Voltage Pulse" {
                n1655 = property class="TabCtl (strict)"(reference=w2327, "Value"=w2326) -> ()  [unwired: 1 in, 2 out]
                n1656 = property class="TabCtl (strict)"(reference=w2327, "Visible"=TRUE) -> ()  [unwired: 1 in, 2 out]
              }
              frame "Jump Train" {
                n1657 = property class="TabCtl (strict)"(reference=w2330, "Value"=w2329) -> ()  [unwired: 1 in, 2 out]
                n1658 = property class="TabCtl (strict)"(reference=w2330, "Visible"=TRUE) -> ()  [unwired: 1 in, 2 out]
              }
              frame "Paired Pulse" {
                n1659 = property class="TabCtl (strict)"(reference=w2333, "Value"=w2332) -> ()  [unwired: 1 in, 2 out]
                n1660 = property class="TabCtl (strict)"(reference=w2333, "Visible"=TRUE) -> ()  [unwired: 1 in, 2 out]
              }
              frame "Single Manip Jump" {
                n1661 = property class="TabCtl (strict)"(reference=w2336, "Value"=w2335) -> ()  [unwired: 1 in, 2 out]
                n1662 = property class="TabCtl (strict)"(reference=w2336, "Visible"=TRUE) -> ()  [unwired: 1 in, 2 out]
              }
              frame "Gap Free" {
                n1663 = property class="TabCtl (strict)"(reference=w2339, "Value"=w2338) -> ()  [unwired: 1 in, 2 out]
                n1664 = property class="TabCtl (strict)"(reference=w2339, "Visible"=TRUE) -> ()  [unwired: 1 in, 2 out]
              }